vi "FlexMag - 24-03-2023.vi"() -> ()   [LabVIEW 2018] (continued)
        n2134 = call-poly <vilib>:"Draw Unflattened Pixmap.vi"("picture"=w2771, "top left point(0, 0)"=cluster{"x":i16, "y":i16} {"x"=204, "y"=150}, "data (RGB format)"=w2772) -> ("new picture"=w2733:picture)  [unwired: 6 in]
        n2135 = call-poly <vilib>:"Draw Unflattened Pixmap.vi"("picture"=w2733, "top left point(0, 0)"=cluster{"x":i16, "y":i16} {"x"=1120, "y"=322}, "data (RGB format)"=w2763) -> ("new picture"=w2734:picture)  [unwired: 6 in]
        n2136 = call-poly <vilib>:"Draw Unflattened Pixmap.vi"("picture"=w2734, "top left point(0, 0)"=cluster{"x":i16, "y":i16} {"x"=794, "y"=322}, "data (RGB format)"=w2764) -> ("new picture"=w2735:picture)  [unwired: 6 in]
        n2137 = call-poly <vilib>:"Draw Unflattened Pixmap.vi"("picture"=w2735, "top left point(0, 0)"=cluster{"x":i16, "y":i16} {"x"=468, "y"=322}, "data (RGB format)"=w2765) -> ("new picture"=w2736:picture)  [unwired: 6 in]
        n2138 = call-poly <vilib>:"Draw Unflattened Pixmap.vi"("picture"=w2736, "top left point(0, 0)"=cluster{"x":i16, "y":i16} {"x"=144, "y"=322}, "data (RGB format)"=w2766) -> ("new picture"=w2697:picture)  [unwired: 6 in]
        n2139 = call-poly <vilib>:"Draw Unflattened Pixmap.vi"("picture"=w2697, "top left point(0, 0)"=cluster{"x":i16, "y":i16} {"x"=1060, "y"=400}, "data (RGB format)"=w2703) -> ("new picture"=w2732:picture)  [unwired: 6 in]
        n2140 = call-poly <vilib>:"Draw Unflattened Pixmap.vi"("picture"=w2732, "top left point(0, 0)"=cluster{"x":i16, "y":i16} {"x"=734, "y"=400}, "data (RGB format)"=w2702) -> ("new picture"=w2731:picture)  [unwired: 6 in]
        n2141 = call-poly <vilib>:"Draw Unflattened Pixmap.vi"("picture"=w2731, "top left point(0, 0)"=cluster{"x":i16, "y":i16} {"x"=408, "y"=400}, "data (RGB format)"=w2701) -> ("new picture"=w2730:picture)  [unwired: 6 in]
        n2142 = call-poly <vilib>:"Draw Unflattened Pixmap.vi"("picture"=w2730, "top left point(0, 0)"=cluster{"x":i16, "y":i16} {"x"=82, "y"=400}, "data (RGB format)"=w2700) -> ("new picture"=w2661:picture)  [unwired: 6 in]
        n2143 = call-poly <vilib>:"Draw Unflattened Pixmap.vi"("picture"=w2661, "top left point(0, 0)"=cluster{"x":i16, "y":i16} {"x"=1117, "y"=398}, "data (RGB format)"=w2691) -> ("new picture"=w2662:picture)  [unwired: 6 in]
        n2144 = call-poly <vilib>:"Draw Unflattened Pixmap.vi"("picture"=w2662, "top left point(0, 0)"=cluster{"x":i16, "y":i16} {"x"=791, "y"=398}, "data (RGB format)"=w2692) -> ("new picture"=w2663:picture)  [unwired: 6 in]
        n2145 = call-poly <vilib>:"Draw Unflattened Pixmap.vi"("picture"=w2663, "top left point(0, 0)"=cluster{"x":i16, "y":i16} {"x"=465, "y"=398}, "data (RGB format)"=w2693) -> ("new picture"=w2664:picture)  [unwired: 6 in]
        n2146 = call-poly <vilib>:"Draw Unflattened Pixmap.vi"("picture"=w2664, "top left point(0, 0)"=cluster{"x":i16, "y":i16} {"x"=139, "y"=398}, "data (RGB format)"=w2694) -> ("new picture"=w2621:picture)  [unwired: 6 in]
        n2147 = call-poly <vilib>:"Draw Unflattened Pixmap.vi"("picture"=w2621, "top left point(0, 0)"=cluster{"x":i16, "y":i16} {"x"=1110, "y"=458}, "data (RGB format)"=w2601) -> ("new picture"=w2659:picture)  [unwired: 6 in]
        n2148 = call-poly <vilib>:"Draw Unflattened Pixmap.vi"("picture"=w2659, "top left point(0, 0)"=cluster{"x":i16, "y":i16} {"x"=784, "y"=458}, "data (RGB format)"=w2630) -> ("new picture"=w2658:picture)  [unwired: 6 in]
        n2149 = call-poly <vilib>:"Draw Unflattened Pixmap.vi"("picture"=w2658, "top left point(0, 0)"=cluster{"x":i16, "y":i16} {"x"=458, "y"=458}, "data (RGB format)"=w2629) -> ("new picture"=w2657:picture)  [unwired: 6 in]
        n2150 = call-poly <vilib>:"Draw Unflattened Pixmap.vi"("picture"=w2657, "top left point(0, 0)"=cluster{"x":i16, "y":i16} {"x"=132, "y"=458}, "data (RGB format)"=w2628) -> ("new picture"=w2602:picture)  [unwired: 6 in]
      }
      frame #1 {
        n2151 = local read "gv bp right fail jpeg"() -> (w3056:u32[][])
        n2152 = local read "gv bp left fail jpeg"() -> (w3028:u32[][])
        n2153 = local read "gv bp right on jpeg"() -> (w3057:u32[][])
        n2154 = local read "gv bp left on jpeg"() -> (w3027:u32[][])
        n2155 = local read "bg bv on jpeg"() -> (w3153:u32[][])
        n2156 = local read "bg bv fail jpeg"() -> (w3152:u32[][])
        n2157 = local read "trns gv fail jpeg"() -> (w3112:u32[][])
        n2158 = local read "ch pg fail jpeg"() -> (w3272:u32[][])
        n2159 = local read "cc fail jpeg"() -> (w3232:u32[][])
        n2160 = local read "ch atm fail jpeg"() -> (w3116:u32[][])
        n2161 = local read "trns gv on jpeg"() -> (w3113:u32[][])
        n2162 = local read "ch pg on jpeg"() -> (w3271:u32[][])
        n2163 = local read "cc on jpeg"() -> (w3233:u32[][])
        n2164 = local read "ch atm on jpeg"() -> (w3115:u32[][])
        n2165 = local read "bg fail jpeg"() -> (w3190:u32[][])
        n2166 = local read "bg on jpeg"() -> (w3191:u32[][])
        n2167 = Build Array(FALSE, "casette_ch1_gui", "casette_ch2_gui", "casette_ch3_gui", "casette_ch4_gui") -> (w3022:bool[])
        n2168 = Build Array(FALSE, "ch2_gv_bp_left_gui", "ch2_gv_bp_left_fail") -> (w3044:bool[])
        n2169 = Build Array(FALSE, "ch3_gv_bp_left_gui", "ch3_gv_bp_left_fail") -> (w3051:bool[])
        n2170 = Build Array(FALSE, "ch1_gv_bp_left_gui", "ch1_gv_bp_left_fail") -> (w3033:bool[])
        n2171 = Build Array(FALSE, "ch3_gv_bp_right_gui", "ch3_gv_bp_right_fail") -> (w3070:bool[])
        n2172 = Build Array(FALSE, "ch4_gv_bp_right_gui", "ch4_gv_bp_right_fail") -> (w3063:bool[])
        n2173 = Build Array(FALSE, "ch4_ch_atm_gui", "ch4_ch_atm_fail") -> (w3133:bool[])
        n2174 = Build Array(FALSE, "ch2_3_trns_gv_gui", "ch2_3_trns_gv_fail") -> (w3100:bool[])
        n2175 = Build Array(FALSE, "ch3_4_trns_gv_gui", "ch3_4_trns_gv_fail") -> (w3107:bool[])
        n2176 = Build Array(FALSE, "ch2_gv_bp_right_gui", "ch2_gv_bp_right_fail") -> (w3081:bool[])
        n2177 = Build Array(FALSE, "ch2_ch_atm_gui", "ch2_ch_atm_fail") -> (w3136:bool[])
        n2178 = Build Array(FALSE, "ch3_ch_atm_gui", "ch3_ch_atm_fail") -> (w3122:bool[])
        n2179 = Build Array(FALSE, "ch1_2_trns_gv_gui", "ch1_2_trns_gv_fail") -> (w3089:bool[])
        n2180 = Build Array(FALSE, "ch4_bg_gui", "ch4_bg_fail") -> (w3209:bool[])
        n2181 = Build Array(FALSE, "ch4_bg_bv_gui", "ch4_bg_bv_fail") -> (w3173:bool[])
        n2182 = Build Array(FALSE, "ch1_ch_atm_gui", "ch1_ch_atm_fail") -> (w3147:bool[])
        n2183 = Build Array(FALSE, "ch2_bg_gui", "ch2_bg_fail") -> (w3212:bool[])
        n2184 = Build Array(FALSE, "ch3_bg_gui", "ch3_bg_fail") -> (w3198:bool[])
        n2185 = Build Array(FALSE, "ch2_bg_bv_gui", "ch2_bg_bv_fail") -> (w3170:bool[])
        n2186 = Build Array(FALSE, "ch3_bg_bv_gui", "ch3_bg_bv_fail") -> (w3184:bool[])
        n2187 = Build Array(FALSE, "ch1_bg_gui", "ch1_bg_fail") -> (w3223:bool[])
        n2188 = Build Array(FALSE, "ch1_bg_bv_gui", "ch1_bg_bv_fail") -> (w3159:bool[])
        n2189 = Build Array(FALSE, "ch4_cc_gui", "ch4_cc_fail") -> (w3249:bool[])
        n2190 = Build Array(FALSE, "ch2_cc_gui", "ch2_cc_fail") -> (w3246:bool[])
        n2191 = Build Array(FALSE, "ch3_cc_gui", "ch3_cc_fail") -> (w3260:bool[])
        n2192 = Build Array(FALSE, "ch4_ch_pg_gui", "ch4_ch_pg_fail") -> (w3286:bool[])
        n2193 = Build Array(FALSE, "ch1_cc_gui", "ch1_cc_fail") -> (w3235:bool[])
        n2194 = Build Array(FALSE, "ch2_ch_pg_gui", "ch2_ch_pg_fail") -> (w3290:bool[])
        n2195 = Build Array(FALSE, "ch3_ch_pg_gui", "ch3_ch_pg_fail") -> (w3275:bool[])
        n2196 = Build Array(FALSE, "ch1_ch_pg_gui", "ch1_ch_pg_fail") -> (w3302:bool[])
        n2197 = property on="Main GUI" class="Pict"() -> ("Mouse"=w3024:T14)  [unwired: 2 in, 2 out]
        n2198 = Boolean Array To Number(Boolean array=w3022) -> (number=w3021:u32)
        n2199 = Boolean Array To Number(Boolean array=w3044) -> (number=w3045:u32)
        n2200 = Boolean Array To Number(Boolean array=w3051) -> (number=w3052:u32)
        n2201 = Boolean Array To Number(Boolean array=w3033) -> (number=w3032:u32)
        n2202 = Boolean Array To Number(Boolean array=w3070) -> (number=w3069:u32)
        n2203 = Boolean Array To Number(Boolean array=w3063) -> (number=w3062:u32)
        n2204 = Boolean Array To Number(Boolean array=w3133) -> (number=w3134:u32)
        n2205 = Boolean Array To Number(Boolean array=w3100) -> (number=w3101:u32)
        n2206 = Boolean Array To Number(Boolean array=w3107) -> (number=w3108:u32)
        n2207 = Boolean Array To Number(Boolean array=w3081) -> (number=w3082:u32)
        n2208 = Boolean Array To Number(Boolean array=w3136) -> (number=w3135:u32)
        n2209 = Boolean Array To Number(Boolean array=w3122) -> (number=w3121:u32)
        n2210 = Boolean Array To Number(Boolean array=w3089) -> (number=w3088:u32)
        n2211 = Boolean Array To Number(Boolean array=w3209) -> (number=w3210:u32)
        n2212 = Boolean Array To Number(Boolean array=w3173) -> (number=w3172:u32)
        n2213 = Boolean Array To Number(Boolean array=w3147) -> (number=w3148:u32)
        n2214 = Boolean Array To Number(Boolean array=w3212) -> (number=w3211:u32)
        n2215 = Boolean Array To Number(Boolean array=w3198) -> (number=w3197:u32)
        n2216 = Boolean Array To Number(Boolean array=w3170) -> (number=w3171:u32)
        n2217 = Boolean Array To Number(Boolean array=w3184) -> (number=w3185:u32)
        n2218 = Boolean Array To Number(Boolean array=w3223) -> (number=w3224:u32)
        n2219 = Boolean Array To Number(Boolean array=w3159) -> (number=w3158:u32)
        n2220 = Boolean Array To Number(Boolean array=w3249) -> (number=w3248:u32)
        n2221 = Boolean Array To Number(Boolean array=w3246) -> (number=w3247:u32)
        n2222 = Boolean Array To Number(Boolean array=w3260) -> (number=w3261:u32)
        n2223 = Boolean Array To Number(Boolean array=w3286) -> (number=w3287:u32)
        n2224 = Boolean Array To Number(Boolean array=w3235) -> (number=w3234:u32)
        n2225 = Boolean Array To Number(Boolean array=w3290) -> (number=w3289:u32)
        n2226 = Boolean Array To Number(Boolean array=w3275) -> (number=w3274:u32)
        n2227 = Boolean Array To Number(Boolean array=w3302) -> (number=w3303:u32)
        n2228 = Mantissa & Exponent(0:w3021) -> (2:w3018:dbl)  [unwired: 1 out]
        n2229 = Mantissa & Exponent(0:w3045) -> (2:w3042:dbl)  [unwired: 1 out]
        n2230 = Mantissa & Exponent(0:w3052) -> (2:w3049:dbl)  [unwired: 1 out]
        n2231 = Mantissa & Exponent(0:w3032) -> (2:w3035:dbl)  [unwired: 1 out]
        n2232 = Mantissa & Exponent(0:w3069) -> (2:w3072:dbl)  [unwired: 1 out]
        n2233 = Mantissa & Exponent(0:w3062) -> (2:w3065:dbl)  [unwired: 1 out]
        n2234 = Mantissa & Exponent(0:w3134) -> (2:w3131:dbl)  [unwired: 1 out]
        n2235 = Mantissa & Exponent(0:w3101) -> (2:w3098:dbl)  [unwired: 1 out]
        n2236 = Mantissa & Exponent(0:w3108) -> (2:w3105:dbl)  [unwired: 1 out]
        n2237 = Mantissa & Exponent(0:w3082) -> (2:w3079:dbl)  [unwired: 1 out]
        n2238 = Mantissa & Exponent(0:w3135) -> (2:w3138:dbl)  [unwired: 1 out]
        n2239 = Mantissa & Exponent(0:w3121) -> (2:w3124:dbl)  [unwired: 1 out]
        n2240 = Mantissa & Exponent(0:w3088) -> (2:w3091:dbl)  [unwired: 1 out]
        n2241 = Mantissa & Exponent(0:w3210) -> (2:w3207:dbl)  [unwired: 1 out]
        n2242 = Mantissa & Exponent(0:w3172) -> (2:w3175:dbl)  [unwired: 1 out]
        n2243 = Mantissa & Exponent(0:w3148) -> (2:w3145:dbl)  [unwired: 1 out]
        n2244 = Mantissa & Exponent(0:w3211) -> (2:w3214:dbl)  [unwired: 1 out]
        n2245 = Mantissa & Exponent(0:w3197) -> (2:w3200:dbl)  [unwired: 1 out]
        n2246 = Mantissa & Exponent(0:w3171) -> (2:w3168:dbl)  [unwired: 1 out]
        n2247 = Mantissa & Exponent(0:w3185) -> (2:w3182:dbl)  [unwired: 1 out]
        n2248 = Mantissa & Exponent(0:w3224) -> (2:w3221:dbl)  [unwired: 1 out]
        n2249 = Mantissa & Exponent(0:w3158) -> (2:w3161:dbl)  [unwired: 1 out]
        n2250 = Mantissa & Exponent(0:w3248) -> (2:w3251:dbl)  [unwired: 1 out]
        n2251 = Mantissa & Exponent(0:w3247) -> (2:w3244:dbl)  [unwired: 1 out]
        n2252 = Mantissa & Exponent(0:w3261) -> (2:w3258:dbl)  [unwired: 1 out]
        n2253 = Mantissa & Exponent(0:w3287) -> (2:w3284:dbl)  [unwired: 1 out]
        n2254 = Mantissa & Exponent(0:w3234) -> (2:w3237:dbl)  [unwired: 1 out]
        n2255 = Mantissa & Exponent(0:w3289) -> (2:w3292:dbl)  [unwired: 1 out]
        n2256 = Mantissa & Exponent(0:w3274) -> (2:w3277:dbl)  [unwired: 1 out]
        n2257 = Mantissa & Exponent(0:w3303) -> (2:w3300:dbl)  [unwired: 1 out]
        n2258 = Unbundle By Name(w3024) -> ("Mouse Position"=→"Mouse Position":cluster{"X":i32, "Y":i32}, "Mouse Modifiers.Button Down"=→"Mouse .Button":bool)
        n2259 = case shown="0, Default" w3042 {
          tunnel: w3027 -> [_ w3318 _]
          tunnel: w3028 -> [_ _ w3319]
          tunnel: [u32[][] [] ("24-bit pixmap") w3318 w3319] -> w3041
          frame 0, Default {
          }
          frame 1 {
          }
          frame 2 {
          }
        }
        n2260 = case shown="0, Default" w3049 {
          tunnel: w3027 -> [_ w3315 _]
          tunnel: w3028 -> [_ _ w3316]
          tunnel: [u32[][] [] ("24-bit pixmap") w3315 w3316] -> w3048
          frame 0, Default {
          }
          frame 1 {
          }
          frame 2 {
          }
        }
        n2261 = case shown="4" w3018 {
          tunnel: [cluster{"x":i16, "y":i16} {"x"=0, "y"=0} ("top left point(0, 0)") cluster{"x":i16, "y":i16} {"x"=1032, "y"=554} ("top left point(0, 0)") cluster{"x":i16, "y":i16} {"x"=708, "y"=554} ("top left point(0, 0)") cluster{"x":i16, "y":i16} {"x"=382, "y"=554} ("top left point(0, 0)") cluster{"x":i16, "y":i16} {"x"=56, "y"=554} ("top left point(0, 0)")] -> w3017
          tunnel: [u32[][] [] ("24-bit pixmap") w3306 w3308 w3310 w3312] -> w3012
          frame 0, Default {
          }
          frame 1 {
            n2262 = local read "casette jpeg"() -> (w3306:u32[][])
          }
          frame 2 {
            n2263 = local read "casette jpeg"() -> (w3308:u32[][])
          }
          frame 3 {
            n2264 = local read "casette jpeg"() -> (w3310:u32[][])
          }
          frame 4 {
            n2265 = local read "casette jpeg"() -> (w3312:u32[][])
          }
        }
        n2266 = case shown="0, Default" w3035 {
          tunnel: w3027 -> [_ w3321 _]
          tunnel: w3028 -> [_ _ w3322]
          tunnel: [u32[][] [] ("24-bit pixmap") w3321 w3322] -> w3036
          frame 0, Default {
          }
          frame 1 {
          }
          frame 2 {
          }
        }
        n2267 = case shown="0, Default" w3072 {
          tunnel: w3057 -> [_ w3327 _]
          tunnel: w3056 -> [_ _ w3328]
          tunnel: [u32[][] [] ("24-bit pixmap") w3327 w3328] -> w3073
          frame 0, Default {
          }
          frame 1 {
          }
          frame 2 {
          }
        }
        n2268 = case shown="0, Default" w3065 {
          tunnel: w3057 -> [_ w3324 _]
          tunnel: w3056 -> [_ _ w3325]
          tunnel: [u32[][] [] ("24-bit pixmap") w3324 w3325] -> w3066
          frame 0, Default {
          }
          frame 1 {
          }
          frame 2 {
          }
        }
        n2269 = case shown="0, Default" w3131 {
          tunnel: w3115 -> [_ w3342 _]
          tunnel: w3116 -> [_ _ w3343]
          tunnel: [u32[][] [] ("24-bit pixmap") w3342 w3343] -> w3130
          frame 0, Default {
          }
          frame 1 {
          }
          frame 2 {
          }
        }
        n2270 = case shown="0, Default" w3098 {
          tunnel: w3113 -> [_ w3336 _]
          tunnel: w3112 -> [_ _ w3337]
          tunnel: [u32[][] [] ("24-bit pixmap") w3336 w3337] -> w3097
          frame 0, Default {
          }
          frame 1 {
          }
          frame 2 {
          }
        }
        n2271 = case shown="0, Default" w3105 {
          tunnel: w3113 -> [_ w3333 _]
          tunnel: w3112 -> [_ _ w3334]
          tunnel: [u32[][] [] ("24-bit pixmap") w3333 w3334] -> w3104
          frame 0, Default {
          }
          frame 1 {
          }
          frame 2 {
          }
        }
        n2272 = case shown="0, Default" w3079 {
          tunnel: w3057 -> [_ w3330 _]
          tunnel: w3056 -> [_ _ w3331]
          tunnel: [u32[][] [] ("24-bit pixmap") w3330 w3331] -> w3078
          frame 0, Default {
          }
          frame 1 {
          }
          frame 2 {
          }
        }
        n2273 = case shown="0, Default" w3138 {
          tunnel: w3115 -> [_ w3348 _]
          tunnel: w3116 -> [_ _ w3349]
          tunnel: [u32[][] [] ("24-bit pixmap") w3348 w3349] -> w3139
          frame 0, Default {
          }
          frame 1 {
          }
          frame 2 {
          }
        }
        n2274 = case shown="0, Default" w3124 {
          tunnel: w3115 -> [_ w3345 _]
          tunnel: w3116 -> [_ _ w3346]
          tunnel: [u32[][] [] ("24-bit pixmap") w3345 w3346] -> w3125
          frame 0, Default {
          }
          frame 1 {
          }
          frame 2 {
          }
        }
        n2275 = case shown="0, Default" w3091 {
          tunnel: w3113 -> [_ w3339 _]
          tunnel: w3112 -> [_ _ w3340]
          tunnel: [u32[][] [] ("24-bit pixmap") w3339 w3340] -> w3092
          frame 0, Default {
          }
          frame 1 {
          }
          frame 2 {
          }
        }
        n2276 = case shown="0, Default" w3207 {
          tunnel: w3191 -> [_ w3366 _]
          tunnel: w3190 -> [_ _ w3367]
          tunnel: [u32[][] [] ("24-bit pixmap") w3366 w3367] -> w3206
          frame 0, Default {
          }
          frame 1 {
          }
          frame 2 {
          }
        }
        n2277 = case shown="0, Default" w3175 {
          tunnel: w3153 -> [_ w3354 _]
          tunnel: w3152 -> [_ _ w3355]
          tunnel: [u32[][] [] ("24-bit pixmap") w3354 w3355] -> w3176
          frame 0, Default {
          }
          frame 1 {
          }
          frame 2 {
          }
        }
        n2278 = case shown="0, Default" w3145 {
          tunnel: w3115 -> [_ w3351 _]
          tunnel: w3116 -> [_ _ w3352]
          tunnel: [u32[][] [] ("24-bit pixmap") w3351 w3352] -> w3144
          frame 0, Default {
          }
          frame 1 {
          }
          frame 2 {
          }
        }
        n2279 = case shown="0, Default" w3214 {
          tunnel: w3191 -> [_ w3372 _]
          tunnel: w3190 -> [_ _ w3373]
          tunnel: [u32[][] [] ("24-bit pixmap") w3372 w3373] -> w3215
          frame 0, Default {
          }
          frame 1 {
          }
          frame 2 {
          }
        }
        n2280 = case shown="0, Default" w3200 {
          tunnel: w3191 -> [_ w3369 _]
          tunnel: w3190 -> [_ _ w3370]
          tunnel: [u32[][] [] ("24-bit pixmap") w3369 w3370] -> w3201
          frame 0, Default {
          }
          frame 1 {
          }
          frame 2 {
          }
        }
        n2281 = case shown="0, Default" w3168 {
          tunnel: w3153 -> [_ w3360 _]
          tunnel: w3152 -> [_ _ w3361]
          tunnel: [u32[][] [] ("24-bit pixmap") w3360 w3361] -> w3167
          frame 0, Default {
          }
          frame 1 {
          }
          frame 2 {
          }
        }
        n2282 = case shown="0, Default" w3182 {
          tunnel: w3153 -> [_ w3357 _]
          tunnel: w3152 -> [_ _ w3358]
          tunnel: [u32[][] [] ("24-bit pixmap") w3357 w3358] -> w3181
          frame 0, Default {
          }
          frame 1 {
          }
          frame 2 {
          }
        }
        n2283 = case shown="0, Default" w3221 {
          tunnel: w3191 -> [_ w3375 _]
          tunnel: w3190 -> [_ _ w3376]
          tunnel: [u32[][] [] ("24-bit pixmap") w3375 w3376] -> w3220
          frame 0, Default {
          }
          frame 1 {
          }
          frame 2 {
          }
        }
        n2284 = case shown="0, Default" w3161 {
          tunnel: w3153 -> [_ w3363 _]
          tunnel: w3152 -> [_ _ w3364]
          tunnel: [u32[][] [] ("24-bit pixmap") w3363 w3364] -> w3162
          frame 0, Default {
          }
          frame 1 {
          }
          frame 2 {
          }
        }
        n2285 = case shown="0, Default" w3251 {
          tunnel: w3233 -> [_ w3378 _]
          tunnel: w3232 -> [_ _ w3379]
          tunnel: [u32[][] [] ("24-bit pixmap") w3378 w3379] -> w3252
          frame 0, Default {
          }
          frame 1 {
          }
          frame 2 {
          }
        }
        n2286 = case shown="0, Default" w3244 {
          tunnel: w3233 -> [_ w3384 _]
          tunnel: w3232 -> [_ _ w3385]
          tunnel: [u32[][] [] ("24-bit pixmap") w3384 w3385] -> w3243
          frame 0, Default {
          }
          frame 1 {
          }
          frame 2 {
          }
        }
        n2287 = case shown="0, Default" w3258 {
          tunnel: w3233 -> [_ w3381 _]
          tunnel: w3232 -> [_ _ w3382]
          tunnel: [u32[][] [] ("24-bit pixmap") w3381 w3382] -> w3257
          frame 0, Default {
          }
          frame 1 {
          }
          frame 2 {
          }
        }
        n2288 = case shown="0, Default" w3284 {
          tunnel: w3271 -> [_ w3390 _]
          tunnel: w3272 -> [_ _ w3391]
          tunnel: [u32[][] [] ("24-bit pixmap") w3390 w3391] -> w3283
          frame 0, Default {
          }
          frame 1 {
          }
          frame 2 {
          }
        }
        n2289 = case shown="0, Default" w3237 {
          tunnel: w3233 -> [_ w3387 _]
          tunnel: w3232 -> [_ _ w3388]
          tunnel: [u32[][] [] ("24-bit pixmap") w3387 w3388] -> w3238
          frame 0, Default {
          }
          frame 1 {
          }
          frame 2 {
          }
        }
        n2290 = case shown="0, Default" w3292 {
          tunnel: w3271 -> [_ w3396 _]
          tunnel: w3272 -> [_ _ w3397]
          tunnel: [u32[][] [] ("24-bit pixmap") w3396 w3397] -> w3293
          frame 0, Default {
          }
          frame 1 {
          }
          frame 2 {
          }
        }
        n2291 = case shown="0, Default" w3277 {
          tunnel: w3271 -> [_ w3393 _]
          tunnel: w3272 -> [_ _ w3394]
          tunnel: [u32[][] [] ("24-bit pixmap") w3393 w3394] -> w3278
          frame 0, Default {
          }
          frame 1 {
          }
          frame 2 {
          }
        }
        n2292 = case shown="0, Default" w3300 {
          tunnel: w3271 -> [_ w3399 _]
          tunnel: w3272 -> [_ _ w3400]
          tunnel: [u32[][] [] ("24-bit pixmap") w3399 w3400] -> w3299
          frame 0, Default {
          }
          frame 1 {
          }
          frame 2 {
          }
        }
        n2293 = call-poly <vilib>:"Draw Unflattened Pixmap.vi"("picture"=w3296, "top left point(0, 0)"=cluster{"x":i16, "y":i16} {"x"=1036, "y"=700}, "data (RGB format)"=w3299) -> ("new picture"=w3288:picture)  [unwired: 6 in]
        n2294 = call-poly <vilib>:"Draw Unflattened Pixmap.vi"("picture"=w3288, "top left point(0, 0)"=cluster{"x":i16, "y":i16} {"x"=712, "y"=700}, "data (RGB format)"=w3293) -> ("new picture"=w3273:picture)  [unwired: 6 in]
        n2295 = call-poly <vilib>:"Draw Unflattened Pixmap.vi"("picture"=w3273, "top left point(0, 0)"=cluster{"x":i16, "y":i16} {"x"=386, "y"=700}, "data (RGB format)"=w3278) -> ("new picture"=w3270:picture)  [unwired: 6 in]
        n2296 = call-poly <vilib>:"Draw Unflattened Pixmap.vi"("picture"=w3270, "top left point(0, 0)"=cluster{"x":i16, "y":i16} {"x"=60, "y"=700}, "data (RGB format)"=w3283) -> ("new picture"=w3229:picture)  [unwired: 6 in]
        n2297 = call-poly <vilib>:"Draw Unflattened Pixmap.vi"("picture"=w3229, "top left point(0, 0)"=cluster{"x":i16, "y":i16} {"x"=1091, "y"=705}, "data (RGB format)"=w3238) -> ("new picture"=w3230:picture)  [unwired: 6 in]
        n2298 = call-poly <vilib>:"Draw Unflattened Pixmap.vi"("picture"=w3230, "top left point(0, 0)"=cluster{"x":i16, "y":i16} {"x"=765, "y"=705}, "data (RGB format)"=w3243) -> ("new picture"=w3231:picture)  [unwired: 6 in]
        n2299 = call-poly <vilib>:"Draw Unflattened Pixmap.vi"("picture"=w3231, "top left point(0, 0)"=cluster{"x":i16, "y":i16} {"x"=439, "y"=705}, "data (RGB format)"=w3257) -> ("new picture"=w3228:picture)  [unwired: 6 in]
        n2300 = call-poly <vilib>:"Draw Unflattened Pixmap.vi"("picture"=w3228, "top left point(0, 0)"=cluster{"x":i16, "y":i16} {"x"=113, "y"=705}, "data (RGB format)"=w3252) -> ("new picture"=w3192:picture)  [unwired: 6 in]
        n2301 = call-poly <vilib>:"Draw Unflattened Pixmap.vi"("picture"=w3192, "top left point(0, 0)"=cluster{"x":i16, "y":i16} {"x"=1164, "y"=754}, "data (RGB format)"=w3220) -> ("new picture"=w3226:picture)  [unwired: 6 in]
        n2302 = call-poly <vilib>:"Draw Unflattened Pixmap.vi"("picture"=w3226, "top left point(0, 0)"=cluster{"x":i16, "y":i16} {"x"=838, "y"=754}, "data (RGB format)"=w3215) -> ("new picture"=w3225:picture)  [unwired: 6 in]
        n2303 = call-poly <vilib>:"Draw Unflattened Pixmap.vi"("picture"=w3225, "top left point(0, 0)"=cluster{"x":i16, "y":i16} {"x"=512, "y"=754}, "data (RGB format)"=w3201) -> ("new picture"=w3227:picture)  [unwired: 6 in]
        n2304 = call-poly <vilib>:"Draw Unflattened Pixmap.vi"("picture"=w3227, "top left point(0, 0)"=cluster{"x":i16, "y":i16} {"x"=186, "y"=754}, "data (RGB format)"=w3206) -> ("new picture"=w3154:picture)  [unwired: 6 in]
        n2305 = call-poly <vilib>:"Draw Unflattened Pixmap.vi"("picture"=w3154, "top left point(0, 0)"=cluster{"x":i16, "y":i16} {"x"=1152, "y"=717}, "data (RGB format)"=w3162) -> ("new picture"=w3156:picture)  [unwired: 6 in]
        n2306 = call-poly <vilib>:"Draw Unflattened Pixmap.vi"("picture"=w3156, "top left point(0, 0)"=cluster{"x":i16, "y":i16} {"x"=826, "y"=717}, "data (RGB format)"=w3167) -> ("new picture"=w3157:picture)  [unwired: 6 in]
        n2307 = call-poly <vilib>:"Draw Unflattened Pixmap.vi"("picture"=w3157, "top left point(0, 0)"=cluster{"x":i16, "y":i16} {"x"=501, "y"=717}, "data (RGB format)"=w3181) -> ("new picture"=w3155:picture)  [unwired: 6 in]
        n2308 = call-poly <vilib>:"Draw Unflattened Pixmap.vi"("picture"=w3155, "top left point(0, 0)"=cluster{"x":i16, "y":i16} {"x"=174, "y"=717}, "data (RGB format)"=w3176) -> ("new picture"=w3114:picture)  [unwired: 6 in]
        n2309 = call-poly <vilib>:"Draw Unflattened Pixmap.vi"("picture"=w3114, "top left point(0, 0)"=cluster{"x":i16, "y":i16} {"x"=1238, "y"=724}, "data (RGB format)"=w3144) -> ("new picture"=w3150:picture)  [unwired: 6 in]
        n2310 = call-poly <vilib>:"Draw Unflattened Pixmap.vi"("picture"=w3150, "top left point(0, 0)"=cluster{"x":i16, "y":i16} {"x"=912, "y"=724}, "data (RGB format)"=w3139) -> ("new picture"=w3149:picture)  [unwired: 6 in]
        n2311 = call-poly <vilib>:"Draw Unflattened Pixmap.vi"("picture"=w3149, "top left point(0, 0)"=cluster{"x":i16, "y":i16} {"x"=586, "y"=724}, "data (RGB format)"=w3125) -> ("new picture"=w3151:picture)  [unwired: 6 in]
        n2312 = call-poly <vilib>:"Draw Unflattened Pixmap.vi"("picture"=w3151, "top left point(0, 0)"=cluster{"x":i16, "y":i16} {"x"=260, "y"=724}, "data (RGB format)"=w3130) -> ("new picture"=w3085:picture)  [unwired: 6 in]
        n2313 = call-poly <vilib>:"Draw Unflattened Pixmap.vi"("picture"=w3085, "top left point(0, 0)"=cluster{"x":i16, "y":i16} {"x"=959, "y"=527}, "data (RGB format)"=w3092) -> ("new picture"=w3086:picture)  [unwired: 6 in]
        n2314 = call-poly <vilib>:"Draw Unflattened Pixmap.vi"("picture"=w3086, "top left point(0, 0)"=cluster{"x":i16, "y":i16} {"x"=633, "y"=527}, "data (RGB format)"=w3097) -> ("new picture"=w3087:picture)  [unwired: 6 in]
        n2315 = call-poly <vilib>:"Draw Unflattened Pixmap.vi"("picture"=w3087, "top left point(0, 0)"=cluster{"x":i16, "y":i16} {"x"=308, "y"=527}, "data (RGB format)"=w3104) -> ("new picture"=w3058:picture)  [unwired: 6 in]
        n2316 = call-poly <vilib>:"Draw Unflattened Pixmap.vi"("picture"=w3058, "top left point(0, 0)"=cluster{"x":i16, "y":i16} {"x"=882, "y"=466}, "data (RGB format)"=w3078) -> ("new picture"=w3084:picture)  [unwired: 6 in]
        n2317 = call-poly <vilib>:"Draw Unflattened Pixmap.vi"("picture"=w3084, "top left point(0, 0)"=cluster{"x":i16, "y":i16} {"x"=556, "y"=466}, "data (RGB format)"=w3073) -> ("new picture"=w3083:picture)  [unwired: 6 in]
        n2318 = call-poly <vilib>:"Draw Unflattened Pixmap.vi"("picture"=w3083, "top left point(0, 0)"=cluster{"x":i16, "y":i16} {"x"=230, "y"=466}, "data (RGB format)"=w3066) -> ("new picture"=w3031:picture)  [unwired: 6 in]
        n2319 = call-poly <vilib>:"Draw Unflattened Pixmap.vi"("picture"=w3031, "top left point(0, 0)"=cluster{"x":i16, "y":i16} {"x"=1042, "y"=466}, "data (RGB format)"=w3036) -> ("new picture"=w3030:picture)  [unwired: 6 in]
        n2320 = call-poly <vilib>:"Draw Unflattened Pixmap.vi"("picture"=w3030, "top left point(0, 0)"=cluster{"x":i16, "y":i16} {"x"=716, "y"=466}, "data (RGB format)"=w3041) -> ("new picture"=w3029:picture)  [unwired: 6 in]
        n2321 = call-poly <vilib>:"Draw Unflattened Pixmap.vi"("picture"=w3029, "top left point(0, 0)"=cluster{"x":i16, "y":i16} {"x"=390, "y"=466}, "data (RGB format)"=w3048) -> ("new picture"=w3020:picture)  [unwired: 6 in]
        n2322 = call-poly <vilib>:"Draw Unflattened Pixmap.vi"("picture"=w3020, "top left point(0, 0)"=w3017, "data (RGB format)"=w3012) -> ("new picture"=w3019:picture)  [unwired: 6 in]
      }
      frame #2 {
        n2323 = local read "trns gv top right fail jpeg"() -> (w3499:u32[][])
        n2324 = local read "trns gv top right on  jpeg"() -> (w3498:u32[][])
        n2325 = local read "trns gv top left on jpeg"() -> (w3488:u32[][])
        n2326 = local read "trns gv top left fail jpeg"() -> (w3487:u32[][])
        n2327 = local read "gv bp right on jpeg"() -> (w3520:u32[][])
        n2328 = local read "gv bp right fail jpeg"() -> (w3521:u32[][])
        n2329 = local read "gv bp left fail jpeg"() -> (w3507:u32[][])
        n2330 = local read "gv bp left on jpeg"() -> (w3508:u32[][])
        n2331 = local read "ch2_gv_bp_right_gui"() -> (w3522:bool)
        n2332 = local read "ch2_gv_bp_right_fail"() -> (w3524:bool)
        n2333 = local read "ch1 front main jpeg"() -> (w3607:u32[][])
        n2334 = local read "ch1_2_trns_gv_gui"() -> (w3486:bool)
        n2335 = local read "ch1_2_trns_gv_fail"() -> (w3484:bool)
        n2336 = local read "ch1_gv_bp_left_gui"() -> (w3455:bool)
        n2337 = local read "ch2_gv_bp_left_gui"() -> (w3506:bool)
        n2338 = local read "ch1_gv_bp_left_fail"() -> (w3454:bool)
        n2339 = local read "ch2_gv_bp_left_fail"() -> (w3504:bool)
        n2340 = local read "ch1_ch_pg_gui"() -> (w3450:bool)
        n2341 = local read "ch1_ch_pg_fail"() -> (w3451:bool)
        n2342 = local read "ch2_3_trns_gv_gui"() -> (w3500:bool)
        n2343 = local read "ch2_3_trns_gv_fail"() -> (w3502:bool)
        n2344 = local read "ch1_bg_bv_gui"() -> (w3448:bool)
        n2345 = local read "ch1_bg_bv_fail"() -> (w3449:bool)
        n2346 = local read "ch1_2_trns_gv_gui"() -> (w3472:bool)
        n2347 = local read "ch1_2_trns_gv_fail"() -> (w3471:bool)
        n2348 = local read "ch1_bg_gui"() -> (w3457:bool)
        n2349 = local read "ch1_bg_fail"() -> (w3456:bool)
        n2350 = local read "trns gv top right fail jpeg"() -> (w3478:u32[][])
        n2351 = local read "sov fail jpeg"() -> (w3592:u32[][])
        n2352 = local read "trns gv top right on  jpeg"() -> (w3475:u32[][])
        n2353 = local read "sov on jpeg"() -> (w3591:u32[][])
        n2354 = local read "ch1_ch_atm_gui"() -> (w3452:bool)
        n2355 = local read "ch1_ch_atm_fail"() -> (w3453:bool)
        n2356 = local read "ch atm on jpeg"() -> (w3542:u32[][])
        n2357 = local read "ch atm fail jpeg"() -> (w3543:u32[][])
        n2358 = local read "ch pg on jpeg"() -> (w3552:u32[][])
        n2359 = local read "ch pg fail jpeg"() -> (w3551:u32[][])
        n2360 = local read "bg bv on jpeg"() -> (w3564:u32[][])
        n2361 = local read "bg bv fail jpeg"() -> (w3565:u32[][])
        n2362 = local read "ch1 top main jpeg"() -> (w3608:u32[][])
        n2363 = local read "cc on jpeg"() -> (w3574:u32[][])
        n2364 = local read "cc fail jpeg"() -> (w3573:u32[][])
        n2365 = local read "bg on jpeg"() -> (w3530:u32[][])
        n2366 = local read "ch2_ch_atm_gui"() -> (w3544:bool)
        n2367 = local read "ch2_ch_atm_fail"() -> (w3546:bool)
        n2368 = local read "bg fail jpeg"() -> (w3529:u32[][])
        n2369 = local read "ch1_cc_gui"() -> (w3446:bool)
        n2370 = local read "ch2_ch_pg_gui"() -> (w3550:bool)
        n2371 = local read "ch1_cc_fail"() -> (w3447:bool)
        n2372 = local read "ch2 front main jpeg"() -> (w3581:u32[][])
        n2373 = local read "ch2_ch_pg_fail"() -> (w3548:bool)
        n2374 = local read "ch2_bg_bv_gui"() -> (w3566:bool)
        n2375 = local read "ch2_bg_bv_fail"() -> (w3568:bool)
        n2376 = local read "ch2_cc_gui"() -> (w3572:bool)
        n2377 = local read "ch2_bg_gui"() -> (w3528:bool)
        n2378 = local read "ch2_cc_fail"() -> (w3570:bool)
        n2379 = local read "ch2_bg_fail"() -> (w3526:bool)
        n2380 = local read "gv bp left fail jpeg"() -> (w3459:u32[][])
        n2381 = local read "gv bp left on jpeg"() -> (w3460:u32[][])
        n2382 = local read "ch atm fail jpeg"() -> (w3431:u32[][])
        n2383 = local read "ch atm on jpeg"() -> (w3432:u32[][])
        n2384 = local read "ch pg fail jpeg"() -> (w3442:u32[][])
        n2385 = local read "bg bv fail jpeg"() -> (w3430:u32[][])
        n2386 = local read "ch pg on jpeg"() -> (w3441:u32[][])
        n2387 = local read "bg bv on jpeg"() -> (w3429:u32[][])
        n2388 = local read "bg fail jpeg"() -> (w3465:u32[][])
        n2389 = local read "sov fail jpeg"() -> (w3593:u32[][])
        n2390 = local read "bg on jpeg"() -> (w3466:u32[][])
        n2391 = local read "sov on jpeg"() -> (w3594:u32[][])
        n2392 = local read "cc fail jpeg"() -> (w3419:u32[][])
        n2393 = local read "ch2 top main jpeg"() -> (w3580:u32[][])
        n2394 = local read "cc on jpeg"() -> (w3420:u32[][])
        n2395 = Build Array(FALSE, "ch2_sov_gui", "ch2_sov_fail") -> (w3585:bool[])
        n2396 = Build Array(FALSE ("element"), w3572, w3570) -> (w3577:bool[])
        n2397 = Build Array(FALSE, w3472, w3471) -> (w3474:bool[])
        n2398 = Build Array(FALSE, w3455, w3454) -> (w3462:bool[])
        n2399 = Build Array(FALSE ("element"), w3528, w3526) -> (w3533:bool[])
        n2400 = Build Array(FALSE ("element"), w3522, w3524) -> (w3517:bool[])
        n2401 = Build Array(FALSE ("element"), w3506, w3504) -> (w3511:bool[])
        n2402 = Build Array(FALSE, w3457, w3456) -> (w3468:bool[])
        n2403 = Build Array(FALSE ("element"), w3550, w3548) -> (w3555:bool[])
        n2404 = Build Array(FALSE ("element"), w3486, w3484) -> (w3490:bool[])
        n2405 = Build Array(FALSE ("element"), w3500, w3502) -> (w3495:bool[])
        n2406 = Build Array(FALSE ("element"), w3544, w3546) -> (w3539:bool[])
        n2407 = Build Array(FALSE, w3452, w3453) -> (w3434:bool[])
        n2408 = Build Array(FALSE ("element"), w3566, w3568) -> (w3561:bool[])
        n2409 = Build Array(FALSE, w3450, w3451) -> (w3439:bool[])
        n2410 = Build Array(FALSE, "ch1_sov_gui", "ch1_sov_fail") -> (w3602:bool[])
        n2411 = Build Array(FALSE, w3448, w3449) -> (w3427:bool[])
        n2412 = Build Array(FALSE, w3446, w3447) -> (w3422:bool[])
        n2413 = Boolean Array To Number(Boolean array=w3585) -> (number=w3584:u32)
        n2414 = Boolean Array To Number(Boolean array=w3577) -> (number=w3578:u32)
        n2415 = Boolean Array To Number(Boolean array=w3533) -> (number=w3534:u32)
        n2416 = Boolean Array To Number(Boolean array=w3517) -> (number=w3516:u32)
        n2417 = Boolean Array To Number(Boolean array=w3511) -> (number=w3512:u32)
        n2418 = Boolean Array To Number(Boolean array=w3555) -> (number=w3556:u32)
        n2419 = Boolean Array To Number(Boolean array=w3490) -> (number=w3491:u32)
        n2420 = Boolean Array To Number(Boolean array=w3495) -> (number=w3494:u32)
        n2421 = Boolean Array To Number(Boolean array=w3474) -> (number=w3473:u32)
        n2422 = Boolean Array To Number(Boolean array=w3539) -> (number=w3538:u32)
        n2423 = Boolean Array To Number(Boolean array=w3561) -> (number=w3560:u32)
        n2424 = Boolean Array To Number(Boolean array=w3462) -> (number=w3463:u32)
        n2425 = Boolean Array To Number(Boolean array=w3468) -> (number=w3469:u32)
        n2426 = Boolean Array To Number(Boolean array=w3434) -> (number=w3435:u32)
        n2427 = Boolean Array To Number(Boolean array=w3439) -> (number=w3438:u32)
        n2428 = Boolean Array To Number(Boolean array=w3602) -> (number=w3603:u32)
        n2429 = Boolean Array To Number(Boolean array=w3427) -> (number=w3426:u32)
        n2430 = Boolean Array To Number(Boolean array=w3422) -> (number=w3423:u32)
        n2431 = Mantissa & Exponent(0:w3584) -> (2:w3588:dbl)  [unwired: 1 out]
        n2432 = Mantissa & Exponent(0:w3578) -> (2:w3576:dbl)  [unwired: 1 out]
        n2433 = Mantissa & Exponent(0:w3473) -> (2:w3477:dbl)  [unwired: 1 out]
        n2434 = Mantissa & Exponent(0:w3463) -> (2:w3461:dbl)  [unwired: 1 out]
        n2435 = Mantissa & Exponent(0:w3534) -> (2:w3532:dbl)  [unwired: 1 out]
        n2436 = Mantissa & Exponent(0:w3516) -> (2:w3518:dbl)  [unwired: 1 out]
        n2437 = Mantissa & Exponent(0:w3512) -> (2:w3510:dbl)  [unwired: 1 out]
        n2438 = Mantissa & Exponent(0:w3469) -> (2:w3467:dbl)  [unwired: 1 out]
        n2439 = Mantissa & Exponent(0:w3556) -> (2:w3554:dbl)  [unwired: 1 out]
        n2440 = Mantissa & Exponent(0:w3491) -> (2:w3489:dbl)  [unwired: 1 out]
        n2441 = Mantissa & Exponent(0:w3494) -> (2:w3496:dbl)  [unwired: 1 out]
        n2442 = Mantissa & Exponent(0:w3538) -> (2:w3540:dbl)  [unwired: 1 out]
        n2443 = Mantissa & Exponent(0:w3435) -> (2:w3433:dbl)  [unwired: 1 out]
        n2444 = Mantissa & Exponent(0:w3560) -> (2:w3562:dbl)  [unwired: 1 out]
        n2445 = Mantissa & Exponent(0:w3438) -> (2:w3440:dbl)  [unwired: 1 out]
        n2446 = Mantissa & Exponent(0:w3603) -> (2:w3599:dbl)  [unwired: 1 out]
        n2447 = Mantissa & Exponent(0:w3426) -> (2:w3428:dbl)  [unwired: 1 out]
        n2448 = Mantissa & Exponent(0:w3423) -> (2:w3421:dbl)  [unwired: 1 out]
        n2449 = case shown="1" w3588 {
          tunnel: w3591 -> [_ w3660 _]
          tunnel: w3592 -> [_ _ w3661]
          tunnel: [u32[][] [] ("24-bit pixmap") w3660 w3661] -> w3583
          frame 0, Default {
          }
          frame 1 {
          }
          frame 2 {
          }
        }
        n2450 = case shown="1" w3576 {
          tunnel: w3574 -> [_ w3657 _]
          tunnel: w3573 -> [_ _ w3658]
          tunnel: [u32[][] [] ("24-bit pixmap") w3657 w3658] -> w3579
          frame 0, Default {
          }
          frame 1 {
          }
          frame 2 {
          }
        }
        n2451 = case shown="2" w3477 {
          tunnel: w3475 -> [_ w3612 _]
          tunnel: w3478 -> [_ _ w3613]
          tunnel: [u32[][] [] ("24-bit pixmap") w3612 w3613] -> w3476
          frame 0, Default {
          }
          frame 1 {
          }
          frame 2 {
          }
        }
        n2452 = case shown="1" w3461 {
          tunnel: w3460 -> [_ w3615 _]
          tunnel: w3459 -> [_ _ w3616]
          tunnel: [u32[][] [] ("24-bit pixmap") w3615 w3616] -> w3464
          frame 0, Default {
          }
          frame 1 {
          }
          frame 2 {
          }
        }
        n2453 = case shown="1" w3532 {
          tunnel: w3530 -> [_ w3645 _]
          tunnel: w3529 -> [_ _ w3646]
          tunnel: [u32[][] [] ("24-bit pixmap") w3645 w3646] -> w3535
          frame 0, Default {
          }
          frame 1 {
          }
          frame 2 {
          }
        }
        n2454 = case shown="1" w3518 {
          tunnel: w3520 -> [_ w3642 _]
          tunnel: w3521 -> [_ _ w3643]
          tunnel: [u32[][] [] ("24-bit pixmap") w3642 w3643] -> w3515
          frame 0, Default {
          }
          frame 1 {
          }
          frame 2 {
          }
        }
        n2455 = case shown="1" w3510 {
          tunnel: w3508 -> [_ w3639 _]
          tunnel: w3507 -> [_ _ w3640]
          tunnel: [u32[][] [] ("24-bit pixmap") w3639 w3640] -> w3513
          frame 0, Default {
          }
          frame 1 {
          }
          frame 2 {
          }
        }
        n2456 = case shown="1" w3467 {
          tunnel: w3466 -> [_ w3618 _]
          tunnel: w3465 -> [_ _ w3619]
          tunnel: [u32[][] [] ("24-bit pixmap") w3618 w3619] -> w3470
          frame 0, Default {
          }
          frame 1 {
          }
          frame 2 {
          }
        }
        n2457 = case shown="1" w3554 {
          tunnel: w3552 -> [_ w3651 _]
          tunnel: w3551 -> [_ _ w3652]
          tunnel: [u32[][] [] ("24-bit pixmap") w3651 w3652] -> w3557
          frame 0, Default {
          }
          frame 1 {
          }
          frame 2 {
          }
        }
        n2458 = case shown="1" w3489 {
          tunnel: w3488 -> [_ w3636 _]
          tunnel: w3487 -> [_ _ w3637]
          tunnel: [u32[][] [] ("24-bit pixmap") w3636 w3637] -> w3492
          frame 0, Default {
          }
          frame 1 {
          }
          frame 2 {
          }
        }
        n2459 = case shown="1" w3496 {
          tunnel: w3498 -> [_ w3633 _]
          tunnel: w3499 -> [_ _ w3634]
          tunnel: [u32[][] [] ("24-bit pixmap") w3633 w3634] -> w3493
          frame 0, Default {
          }
          frame 1 {
          }
          frame 2 {
          }
        }
        n2460 = case shown="1" w3540 {
          tunnel: w3542 -> [_ w3648 _]
          tunnel: w3543 -> [_ _ w3649]
          tunnel: [u32[][] [] ("24-bit pixmap") w3648 w3649] -> w3537
          frame 0, Default {
          }
          frame 1 {
          }
          frame 2 {
          }
        }
        n2461 = case shown="1" w3433 {
          tunnel: w3432 -> [_ w3621 _]
          tunnel: w3431 -> [_ _ w3622]
          tunnel: [u32[][] [] ("24-bit pixmap") w3621 w3622] -> w3436
          frame 0, Default {
          }
          frame 1 {
          }
          frame 2 {
          }
        }
        n2462 = case shown="1" w3562 {
          tunnel: w3564 -> [_ w3654 _]
          tunnel: w3565 -> [_ _ w3655]
          tunnel: [u32[][] [] ("24-bit pixmap") w3654 w3655] -> w3559
          frame 0, Default {
          }
          frame 1 {
          }
          frame 2 {
          }
        }
        n2463 = case shown="1" w3440 {
          tunnel: w3441 -> [_ w3624 _]
          tunnel: w3442 -> [_ _ w3625]
          tunnel: [u32[][] [] ("24-bit pixmap") w3624 w3625] -> w3437
          frame 0, Default {
          }
          frame 1 {
          }
          frame 2 {
          }
        }
        n2464 = case shown="1" w3599 {
          tunnel: w3594 -> [_ w3663 _]
          tunnel: w3593 -> [_ _ w3664]
          tunnel: [u32[][] [] ("24-bit pixmap") w3663 w3664] -> w3604
          frame 0, Default {
          }
          frame 1 {
          }
          frame 2 {
          }
        }
        n2465 = case shown="1" w3428 {
          tunnel: w3429 -> [_ w3627 _]
          tunnel: w3430 -> [_ _ w3628]
          tunnel: [u32[][] [] ("24-bit pixmap") w3627 w3628] -> w3425
          frame 0, Default {
          }
          frame 1 {
          }
          frame 2 {
          }
        }
        n2466 = case shown="1" w3421 {
          tunnel: w3420 -> [_ w3630 _]
          tunnel: w3419 -> [_ _ w3631]
          tunnel: [u32[][] [] ("24-bit pixmap") w3630 w3631] -> w3424
          frame 0, Default {
          }
          frame 1 {
          }
          frame 2 {
          }
        }
        n2467 = call-poly <vilib>:"Draw Unflattened Pixmap.vi"("top left point(0, 0)"=cluster{"x":i16, "y":i16} {"x"=80, "y"=180}, "data (RGB format)"=w3580) -> ("new picture"=w3582:picture)  [unwired: 7 in]
        n2468 = call-poly <vilib>:"Draw Unflattened Pixmap.vi"("top left point(0, 0)"=cluster{"x":i16, "y":i16} {"x"=80, "y"=180}, "data (RGB format)"=w3581) -> ("new picture"=→"CH2 front main":picture)  [unwired: 7 in]
        n2469 = call-poly <vilib>:"Draw Unflattened Pixmap.vi"("top left point(0, 0)"=cluster{"x":i16, "y":i16} {"x"=80, "y"=180}, "data (RGB format)"=w3607) -> ("new picture"=→"CH1 front main":picture)  [unwired: 7 in]
        n2470 = call-poly <vilib>:"Draw Unflattened Pixmap.vi"("top left point(0, 0)"=cluster{"x":i16, "y":i16} {"x"=80, "y"=180}, "data (RGB format)"=w3608) -> ("new picture"=w3595:picture)  [unwired: 7 in]
        n2471 = call-poly <vilib>:"Draw Unflattened Pixmap.vi"("picture"=w3582, "top left point(0, 0)"=cluster{"x":i16, "y":i16} {"x"=492, "y"=218}, "data (RGB format)"=w3583) -> ("new picture"=w3569:picture)  [unwired: 6 in]
        n2472 = call-poly <vilib>:"Draw Unflattened Pixmap.vi"("picture"=w3569, "top left point(0, 0)"=cluster{"x":i16, "y":i16} {"x"=258, "y"=636}, "data (RGB format)"=w3579) -> ("new picture"=w3558:picture)  [unwired: 6 in]
        n2473 = call-poly <vilib>:"Draw Unflattened Pixmap.vi"("picture"=w3558, "top left point(0, 0)"=cluster{"x":i16, "y":i16} {"x"=350, "y"=648}, "data (RGB format)"=w3559) -> ("new picture"=w3547:picture)  [unwired: 6 in]
        n2474 = call-poly <vilib>:"Draw Unflattened Pixmap.vi"("picture"=w3547, "top left point(0, 0)"=cluster{"x":i16, "y":i16} {"x"=184, "y"=632}, "data (RGB format)"=w3557) -> ("new picture"=w3536:picture)  [unwired: 6 in]
        n2475 = call-poly <vilib>:"Draw Unflattened Pixmap.vi"("picture"=w3536, "top left point(0, 0)"=cluster{"x":i16, "y":i16} {"x"=464, "y"=654}, "data (RGB format)"=w3537) -> ("new picture"=w3525:picture)  [unwired: 6 in]
        n2476 = call-poly <vilib>:"Draw Unflattened Pixmap.vi"("picture"=w3525, "top left point(0, 0)"=cluster{"x":i16, "y":i16} {"x"=362, "y"=686}, "data (RGB format)"=w3535) -> ("new picture"=w3514:picture)  [unwired: 6 in]
        n2477 = call-poly <vilib>:"Draw Unflattened Pixmap.vi"("picture"=w3514, "top left point(0, 0)"=cluster{"x":i16, "y":i16} {"x"=474, "y"=298}, "data (RGB format)"=w3515) -> ("new picture"=w3503:picture)  [unwired: 6 in]
        n2478 = call-poly <vilib>:"Draw Unflattened Pixmap.vi"("picture"=w3503, "top left point(0, 0)"=cluster{"x":i16, "y":i16} {"x"=160, "y"=298}, "data (RGB format)"=w3513) -> ("new picture"=w3481:picture)  [unwired: 6 in]
        n2479 = call-poly <vilib>:"Draw Unflattened Pixmap.vi"("picture"=w3481, "top left point(0, 0)"=cluster{"x":i16, "y":i16} {"x"=554, "y"=362}, "data (RGB format)"=w3492) -> ("new picture"=w3482:picture)  [unwired: 6 in]
        n2480 = call-poly <vilib>:"Draw Unflattened Pixmap.vi"("picture"=w3482, "top left point(0, 0)"=cluster{"x":i16, "y":i16} {"x"=80, "y"=360}, "data (RGB format)"=w3493) -> ("new picture"=→"CH2 top main":picture)  [unwired: 6 in]
        n2481 = call-poly <vilib>:"Draw Unflattened Pixmap.vi"("picture"=w3595, "top left point(0, 0)"=cluster{"x":i16, "y":i16} {"x"=492, "y"=218}, "data (RGB format)"=w3604) -> ("new picture"=w3402:picture)  [unwired: 6 in]
        n2482 = call-poly <vilib>:"Draw Unflattened Pixmap.vi"("picture"=w3402, "top left point(0, 0)"=cluster{"x":i16, "y":i16} {"x"=258, "y"=636}, "data (RGB format)"=w3424) -> ("new picture"=w3444:picture)  [unwired: 6 in]
        n2483 = call-poly <vilib>:"Draw Unflattened Pixmap.vi"("picture"=w3444, "top left point(0, 0)"=cluster{"x":i16, "y":i16} {"x"=350, "y"=648}, "data (RGB format)"=w3425) -> ("new picture"=w3443:picture)  [unwired: 6 in]
        n2484 = call-poly <vilib>:"Draw Unflattened Pixmap.vi"("picture"=w3443, "top left point(0, 0)"=cluster{"x":i16, "y":i16} {"x"=184, "y"=632}, "data (RGB format)"=w3437) -> ("new picture"=w3445:picture)  [unwired: 6 in]
        n2485 = call-poly <vilib>:"Draw Unflattened Pixmap.vi"("picture"=w3445, "top left point(0, 0)"=cluster{"x":i16, "y":i16} {"x"=464, "y"=654}, "data (RGB format)"=w3436) -> ("new picture"=w3418:picture)  [unwired: 6 in]
        n2486 = call-poly <vilib>:"Draw Unflattened Pixmap.vi"("picture"=w3418, "top left point(0, 0)"=cluster{"x":i16, "y":i16} {"x"=362, "y"=684}, "data (RGB format)"=w3470) -> ("new picture"=w3458:picture)  [unwired: 6 in]
        n2487 = call-poly <vilib>:"Draw Unflattened Pixmap.vi"("picture"=w3458, "top left point(0, 0)"=cluster{"x":i16, "y":i16} {"x"=166, "y"=298}, "data (RGB format)"=w3464) -> ("new picture"=w3417:picture)  [unwired: 6 in]
        n2488 = call-poly <vilib>:"Draw Unflattened Pixmap.vi"("picture"=w3417, "top left point(0, 0)"=cluster{"x":i16, "y":i16} {"x"=80, "y"=362}, "data (RGB format)"=w3476) -> ("new picture"=→"CH1 top main":picture)  [unwired: 6 in]
      }
      frame #3 {
        n2489 = local read "ch4_gv_bp_right_gui"() -> (w3714:bool)
        n2490 = local read "ch4_gv_bp_right_fail"() -> (w3713:bool)
        n2491 = local read "ch4_ch_pg_gui"() -> (w3709:bool)
        n2492 = local read "ch4_ch_pg_fail"() -> (w3710:bool)
        n2493 = local read "ch4_bg_bv_gui"() -> (w3707:bool)
        n2494 = local read "ch4_bg_bv_fail"() -> (w3708:bool)
        n2495 = local read "ch3_4_trns_gv_gui"() -> (w3734:bool)
        n2496 = local read "ch3_4_trns_gv_fail"() -> (w3733:bool)
        n2497 = local read "ch3_gv_bp_right_gui"() -> (w3795:bool)
        n2498 = local read "ch3_gv_bp_right_fail"() -> (w3796:bool)
        n2499 = local read "ch4_bg_gui"() -> (w3716:bool)
        n2500 = local read "ch4_bg_fail"() -> (w3715:bool)
        n2501 = local read "ch3_ch_pg_gui"() -> (w3802:bool)
        n2502 = local read "ch3_ch_pg_fail"() -> (w3801:bool)
        n2503 = local read "ch4_ch_atm_gui"() -> (w3711:bool)
        n2504 = local read "ch4_ch_atm_fail"() -> (w3712:bool)
        n2505 = local read "ch3_bg_bv_gui"() -> (w3804:bool)
        n2506 = local read "ch3_gv_bp_left_gui"() -> (w3797:bool)
        n2507 = local read "trns gv top left fail jpeg"() -> (w3742:u32[][])
        n2508 = local read "ch3_bg_bv_fail"() -> (w3803:bool)
        n2509 = local read "ch3_gv_bp_left_fail"() -> (w3798:bool)
        n2510 = local read "ch3_4_trns_gv_gui"() -> (w3753:bool)
        n2511 = local read "ch3_4_trns_gv_fail"() -> (w3754:bool)
        n2512 = local read "trns gv top left on jpeg"() -> (w3738:u32[][])
        n2513 = local read "ch2_3_trns_gv_gui"() -> (w3757:bool)
        n2514 = local read "ch2_3_trns_gv_fail"() -> (w3756:bool)
        n2515 = local read "ch3_bg_gui"() -> (w3793:bool)
        n2516 = local read "ch3_bg_fail"() -> (w3794:bool)
        n2517 = local read "trns gv top right fail jpeg"() -> (w3743:u32[][])
        n2518 = local read "trns gv top right on  jpeg"() -> (w3749:u32[][])
        n2519 = local read "ch3_ch_atm_gui"() -> (w3800:bool)
        n2520 = local read "ch3_ch_atm_fail"() -> (w3799:bool)
        n2521 = local read "ch4_cc_gui"() -> (w3705:bool)
        n2522 = local read "ch4_cc_fail"() -> (w3706:bool)
        n2523 = local read "ch3_cc_gui"() -> (w3806:bool)
        n2524 = local read "ch3_cc_fail"() -> (w3805:bool)
        n2525 = local read "trns gv top left fail jpeg"() -> (w3764:u32[][])
        n2526 = local read "trns gv top left on jpeg"() -> (w3763:u32[][])
        n2527 = local read "gv bp right fail jpeg"() -> (w3721:u32[][])
        n2528 = local read "gv bp right on jpeg"() -> (w3722:u32[][])
        n2529 = local read "gv bp left fail jpeg"() -> (w3775:u32[][])
        n2530 = local read "gv bp left on jpeg"() -> (w3776:u32[][])
        n2531 = local read "gv bp right fail jpeg"() -> (w3786:u32[][])
        n2532 = local read "gv bp right on jpeg"() -> (w3785:u32[][])
        n2533 = local read "ch atm fail jpeg"() -> (w3685:u32[][])
        n2534 = local read "ch atm on jpeg"() -> (w3686:u32[][])
        n2535 = local read "ch pg fail jpeg"() -> (w3696:u32[][])
        n2536 = local read "bg bv fail jpeg"() -> (w3682:u32[][])
        n2537 = local read "ch pg on jpeg"() -> (w3695:u32[][])
        n2538 = local read "bg bv on jpeg"() -> (w3681:u32[][])
        n2539 = local read "bg fail jpeg"() -> (w3727:u32[][])
        n2540 = local read "ch atm fail jpeg"() -> (w3826:u32[][])
        n2541 = local read "bg on jpeg"() -> (w3728:u32[][])
        n2542 = local read "sov fail jpeg"() -> (w3859:u32[][])
        n2543 = local read "ch atm on jpeg"() -> (w3825:u32[][])
        n2544 = local read "sov on jpeg"() -> (w3858:u32[][])
        n2545 = local read "cc fail jpeg"() -> (w3671:u32[][])
        n2546 = local read "ch pg fail jpeg"() -> (w3815:u32[][])
        n2547 = local read "bg bv fail jpeg"() -> (w3829:u32[][])
        n2548 = local read "cc on jpeg"() -> (w3672:u32[][])
        n2549 = local read "ch pg on jpeg"() -> (w3816:u32[][])
        n2550 = local read "bg bv on jpeg"() -> (w3830:u32[][])
        n2551 = local read "bg fail jpeg"() -> (w3772:u32[][])
        n2552 = local read "sov fail jpeg"() -> (w3861:u32[][])
        n2553 = local read "bg on jpeg"() -> (w3771:u32[][])
        n2554 = local read "sov on jpeg"() -> (w3862:u32[][])
        n2555 = local read "ch4 front main jpeg"() -> (w3872:u32[][])
        n2556 = local read "cc fail jpeg"() -> (w3841:u32[][])
        n2557 = local read "cc on jpeg"() -> (w3840:u32[][])
        n2558 = local read "ch4 top main jpeg"() -> (w3871:u32[][])
        n2559 = local read "ch3 top main jpeg"() -> (w3873:u32[][])
        n2560 = Build Array(FALSE, w3734, w3733) -> (w3737:bool[])
        n2561 = local read "ch3 front main jpeg"() -> (w3874:u32[][])
        n2562 = Build Array(FALSE, w3714, w3713) -> (w3724:bool[])
        n2563 = Build Array(FALSE, w3716, w3715) -> (w3730:bool[])
        n2564 = Build Array(FALSE, w3711, w3712) -> (w3688:bool[])
        n2565 = Build Array(FALSE, w3709, w3710) -> (w3693:bool[])
        n2566 = Build Array(FALSE, w3707, w3708) -> (w3679:bool[])
        n2567 = Build Array(FALSE, w3705, w3706) -> (w3674:bool[])
        n2568 = Build Array(FALSE, "ch4_sov_gui", "ch4_sov_fail") -> (w3854:bool[])
        n2569 = Build Array(FALSE, w3753, w3754) -> (w3750:bool[])
        n2570 = Build Array(FALSE, w3797, w3798) -> (w3778:bool[])
        n2571 = Build Array(FALSE, w3757, w3756) -> (w3761:bool[])
        n2572 = Build Array(FALSE, w3795, w3796) -> (w3783:bool[])
        n2573 = Build Array(FALSE, w3793, w3794) -> (w3769:bool[])
        n2574 = Build Array(FALSE, w3800, w3799) -> (w3823:bool[])
        n2575 = Build Array(FALSE, w3802, w3801) -> (w3818:bool[])
        n2576 = Build Array(FALSE, "ch3_sov_gui", "ch3_sov_fail") -> (w3866:bool[])
        n2577 = Build Array(FALSE, w3804, w3803) -> (w3832:bool[])
        n2578 = Build Array(FALSE, w3806, w3805) -> (w3838:bool[])
        n2579 = Boolean Array To Number(Boolean array=w3737) -> (number=w3736:u32)
        n2580 = Boolean Array To Number(Boolean array=w3724) -> (number=w3725:u32)
        n2581 = Boolean Array To Number(Boolean array=w3730) -> (number=w3731:u32)
        n2582 = Boolean Array To Number(Boolean array=w3688) -> (number=w3689:u32)
        n2583 = Boolean Array To Number(Boolean array=w3693) -> (number=w3692:u32)
        n2584 = Boolean Array To Number(Boolean array=w3679) -> (number=w3678:u32)
        n2585 = Boolean Array To Number(Boolean array=w3854) -> (number=w3853:u32)
        n2586 = Boolean Array To Number(Boolean array=w3674) -> (number=w3675:u32)
        n2587 = Boolean Array To Number(Boolean array=w3750) -> (number=w3751:u32)
        n2588 = Boolean Array To Number(Boolean array=w3778) -> (number=w3779:u32)
        n2589 = Boolean Array To Number(Boolean array=w3761) -> (number=w3760:u32)
        n2590 = Boolean Array To Number(Boolean array=w3783) -> (number=w3782:u32)
        n2591 = Boolean Array To Number(Boolean array=w3769) -> (number=w3768:u32)
        n2592 = Boolean Array To Number(Boolean array=w3823) -> (number=w3822:u32)
        n2593 = Boolean Array To Number(Boolean array=w3818) -> (number=w3819:u32)
        n2594 = Boolean Array To Number(Boolean array=w3866) -> (number=w3867:u32)
        n2595 = Boolean Array To Number(Boolean array=w3832) -> (number=w3833:u32)
        n2596 = Boolean Array To Number(Boolean array=w3838) -> (number=w3837:u32)
        n2597 = Mantissa & Exponent(0:w3736) -> (2:w3741:dbl)  [unwired: 1 out]
        n2598 = Mantissa & Exponent(0:w3725) -> (2:w3723:dbl)  [unwired: 1 out]
        n2599 = Mantissa & Exponent(0:w3731) -> (2:w3729:dbl)  [unwired: 1 out]
        n2600 = Mantissa & Exponent(0:w3689) -> (2:w3687:dbl)  [unwired: 1 out]
        n2601 = Mantissa & Exponent(0:w3692) -> (2:w3694:dbl)  [unwired: 1 out]
        n2602 = Mantissa & Exponent(0:w3678) -> (2:w3680:dbl)  [unwired: 1 out]
        n2603 = Mantissa & Exponent(0:w3853) -> (2:w3857:dbl)  [unwired: 1 out]
        n2604 = Mantissa & Exponent(0:w3675) -> (2:w3673:dbl)  [unwired: 1 out]
        n2605 = Mantissa & Exponent(0:w3751) -> (2:w3744:dbl)  [unwired: 1 out]
        n2606 = Mantissa & Exponent(0:w3779) -> (2:w3777:dbl)  [unwired: 1 out]
        n2607 = Mantissa & Exponent(0:w3760) -> (2:w3762:dbl)  [unwired: 1 out]